vi "Main.vi"() -> ()   [LabVIEW 2018] (continued)
  # "(Shutter Off)"
  # "V_IF (0.5pi or -1.5pi)"
  # "V_IF (pi or -pi)"
  # "V_IF (1.5pi or -0.5pi)"
  # "Pixel width calibration:\n1. Move the cursor to a feature pixel that you can recognize\n2. Click \"Record X1\" to record the X coordinate\n\n \n3. Use \"X-\" or \"X+\" with \"XY Step\" of 30 um to move the image horizentally by 30 um\n4. Move the cursor to the same feature pixel\n5. Click \"Record X2\" to record the X coordinate again\n\n\n6. Click \"Pixel Width\" to calculate the pixel width (um/px)\n7. Input your desired pixel width (um/px) and the cooresponding \"XY Factor (1/V)\" will be calculated"
  # "Based on \"Desired Pixel Wdith (um)\""
  # "Going inside the sample (Z increase)"
  # "Z4\nAst45"
  # "Z5\nDef"
  # "Z6\nAst0"
  # "Z7\nTreY"
  # "Z8\nComX"
  # "Z9\nComY"
  # "Z10\nTreX"
  # "Z11\nTetY"
  # "Z12\nSAstY"
  # "Z13\nSAb3"
  # "Z14\nSAstX"
  # "Z15\nTetX"
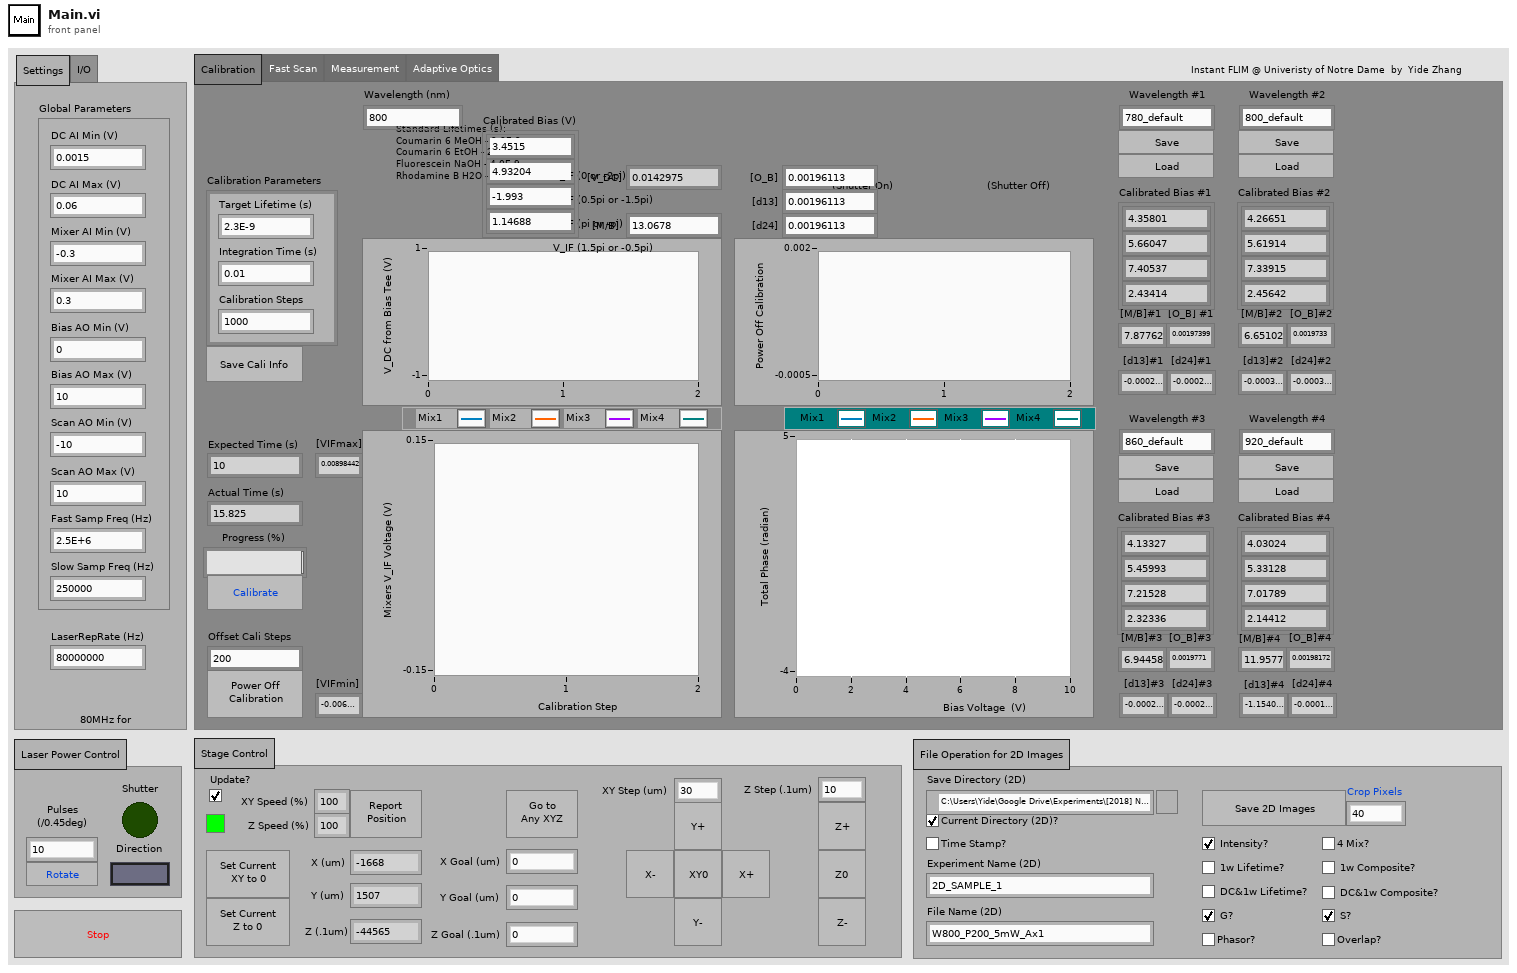
[diagram p1: front panel]
types:
  T1 = cluster{"DC AI Min (V)":dbl, "DC AI Max (V)":dbl, "Mixer AI Min (V)":dbl, "Mixer AI Max (V)":dbl, "Bias AO Min (V)":dbl, "Bias AO Max (V)":dbl, "Scan AO Min (V)":dbl, "Scan AO Max (V)":dbl, "Fast Samp Freq (Hz)":dbl, "Slow Samp Freq (Hz)":dbl}
  T2 = enum32{"Calibration", "Fast Scan", "Measurement", "Adaptive Optics"}
  T3 = cluster{"Target Lifetime (s)":dbl, "Integration Time (s)":dbl, "Calibration Steps":dbl}
  T4 = cluster{"Pixel Dwell Time (s)":dbl, "Pixel Size":dbl, "X Min (V)":dbl, "X Max (V)":dbl, "Y Min (V)":dbl, "Y Max (V)":dbl, "XY Factor (1/V)":dbl}
  T5 = enum16{"Nikon 40X NA 0.8 WD=3.5mm", "Olympus 25X NA 1.05 WD=2mm"}
  T6 = enum32{"Process", "Results", "Phasors", "Z-Stack", "Time-Lapse", "GSOS Process", "GSOS Results"}
  T7 = cluster{"X Values":dbl[], "Histogram: h(x)":i32[]}
  T8 = enum16{"fire", "rainbow", "gray", "inverse gray", "ice", "original"}
  T9 = cluster{bool[], dbl[], cluster{dbl, dbl}[], u32[]}
  T10 = enum16{"Intensity 3D", "1w Lifetime 3D", "DC&1w Lifetime 3D", "1w Composite 3D", "DC&1w Composite 3D", "Phasor 3D", "Overlap 3D"}
  T11 = enum16{"Mean Pixel Value", "Normalized Variance", "Mean Squared Pixel Value"}
  T12 = cluster{"Mixer AI Channel(s)":tag, "DC AI Channel(s)":tag, "Bias AO Channel(s) ":tag, "Scan AO Channel(s)":tag}
  T13 = enum32{"Calibration", "Fast Scan", "Measurement"}
  T14 = cluster{"DC AI task out":refnum<k21>, "Mixer AI task out":refnum<k21>, "Bias AO task out":refnum<k21>, "Scan AO task out":refnum<k21>}
  T15 = typedef "NI_LVConfig.lvlib/Config Data RefNum.ctl" = refnum<k1>
  T16 = typedef "LVBoundsTypeDef.ctl" = cluster{"Width":u32, "Height":u32}
  T17 = typedef "lveventtype.ctl" = enum32{"Null", "Timeout", "Annotation Menu Selection", "Annotation Menu Selection?", "App Instance Close", "App Instance Close?", "Autoscale Range Change", "Bookmark Info Change", "Cell Edit", "Cell Edit?", "Cursor Grab", "Cursor Grab?", "Cursor Menu Selection", "Cursor Menu Selection?", "Cursor Move", "Cursor Release", "Data Change", "Direction Change", "Display State Change", "Drag Ended", "Drag Enter", "Drag Leave", "Drag Over", "Drag Source Update", "Drag Starting", "Drag Starting?", "Drop", "Exec State Change", "Key Down", "Key Down?", "Key Repeat", "Key Repeat?", "Key Up", "Listbox Double Click", "Menu Activation?", "Menu Selection (App)", "Menu Selection? (App)", "Menu Selection (User)", "Mouse Down", "Mouse Down?", "Mouse Enter", "Mouse Leave", "Mouse Move", "Mouse Up", "Mouse Wheel", "NI Security User Change (App)", "Pane Size", "Panel Close", "Panel Close?", "Panel Resize", "Plot Attribute Change", "Scale Range Change", "Shortcut Menu Activation?", "Shortcut Menu Selection (App)", "Shortcut Menu Selection? (App)", "Shortcut Menu Selection (User)", "Tree Double Click", "Tree Drag", "Tree Drag?", "Tree Drop", "Tree Drop?", "Tree Item Close", "Tree Item Close?", "Tree Item Open", "Tree Item Open?", "User Event", "Value Change"}
  T18 = typedef "LVRectTypeDef.ctl" = cluster{"Left":i16, "Top":i16, "Right":i16, "Bottom":i16}
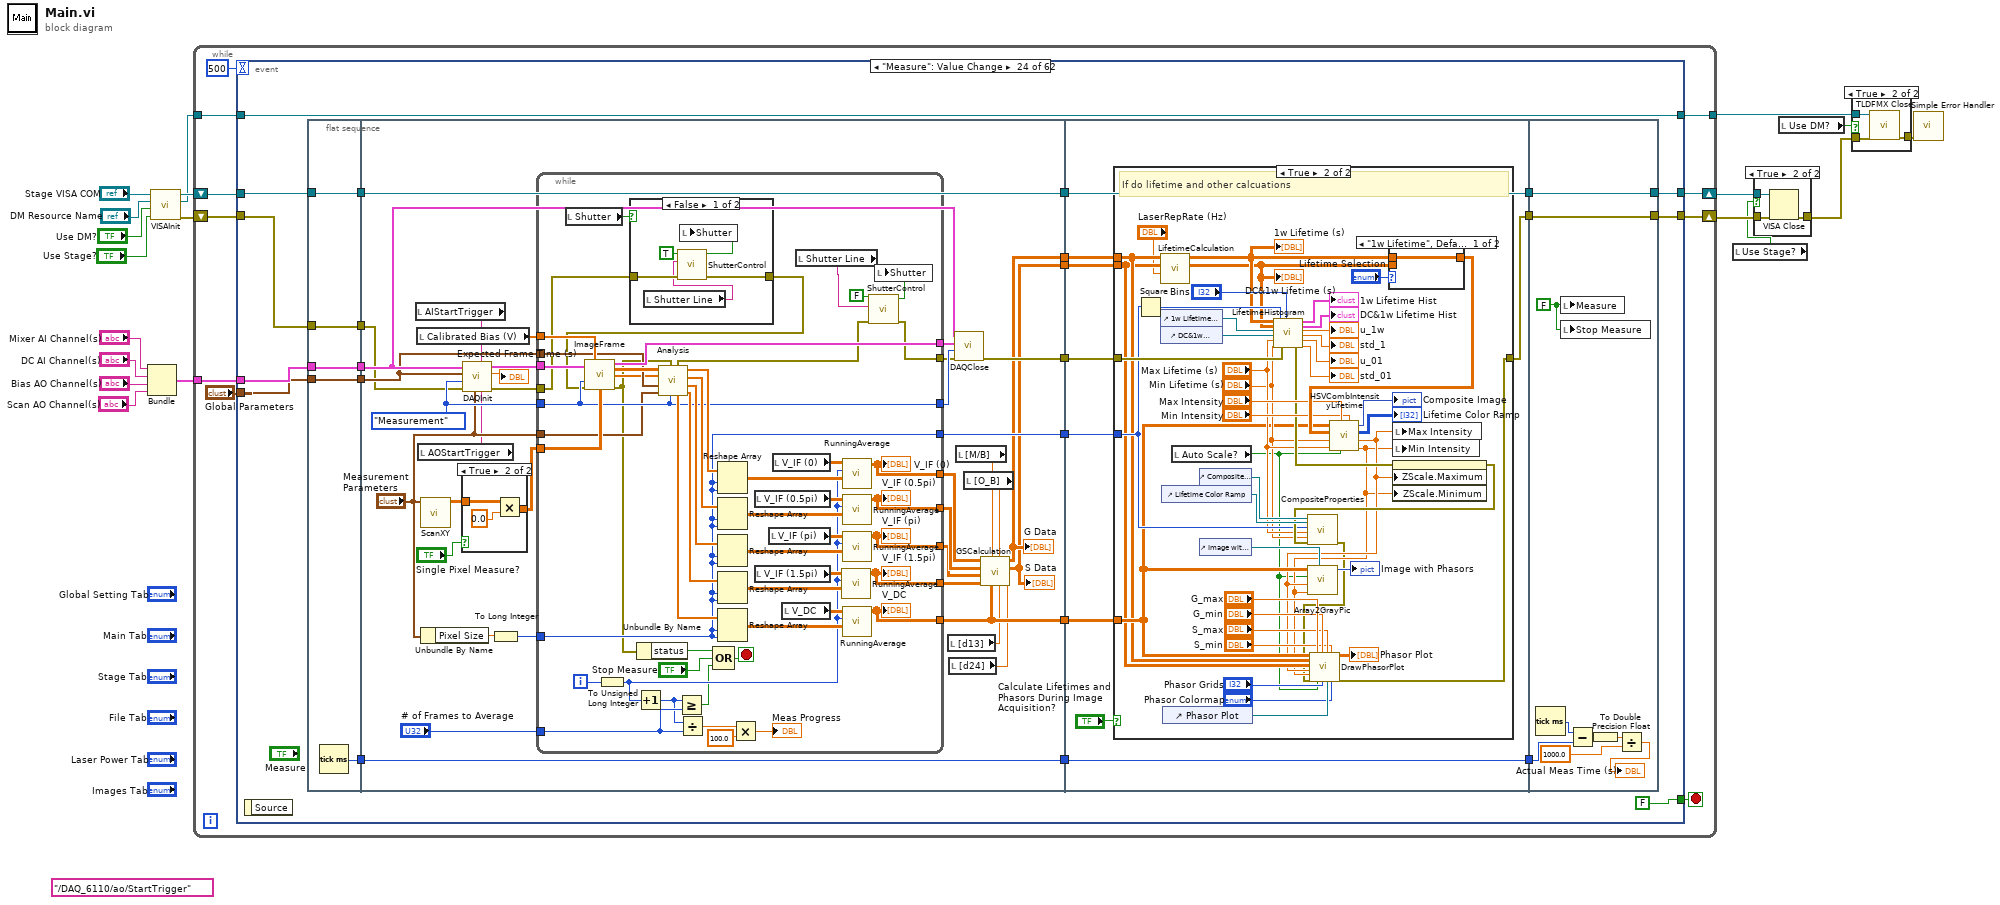
[diagram p0: block diagram]
diagram:
  (unwired) tag "/DAQ_6110/ao/StartTrigger" ("source")
  n1 = Bundle("Mixer AI Channel(s)"="Mixer AI Channel(s)", "DC AI Channel(s)"="DC AI Channel(s)", "Bias AO Channel(s)"="Bias AO Channel(s)", "Scan AO Channel(s)"="Scan AO Channel(s)") -> (w15:T12)  [unwired: 1 in]
  n2 = call "VISAInit.vi"("Use Stage?"="Use Stage?", "Use DM?"="Use DM?", "DM Resource Name"="DM Resource Name", "Stage Resource Name"="Stage VISA COM") -> ("error out"=w14:errorcluster, "DM Handle"=w10:refnum<visa-resource-name>, "Stage Resource"=w13:refnum<visa-resource-name>)  [unwired: 5 in]
  n3 = while {
    shift-right: [w24] -> w19
    shift-left: w13 -> [w29]
    shift-right: [w23] -> w18
    shift-left: w14 -> [w28]
    tunnel: w15 -> [w27]
    tunnel: w10 -> [w22]
    tunnel: [w21] -> w7
    stop <- w26 stop-if-true
    n4 = event shown="[23] \"Measure\": Value Change" {
      selector: _ -> [_ _ _ _ _ _ _ _ _ _ _ _ _ _ _ _ _ _ _ _ _ _ _ _ _ _ _ _ _ _ _ _ _ _ _ _ _ _ _ _ _ _ _ _ _ _ _ _ _ _ _ _ _ _ _ _ _ _ _ _ _ _]
      dyn-events: _ -> [_ _ _ _ _ _ _ _ _ _ _ _ _ _ _ _ _ _ _ _ _ _ _ _ _ _ _ _ _ _ _ _ _ _ _ _ _ _ _ _ _ _ _ _ _ _ _ _ _ _ _ _ _ _ _ _ _ _ _ _ _ _]
      timeout: 500 -> [_ _ _ _ _ _ _ _ _ _ _ _ _ _ _ _ _ _ _ _ _ _ _ _ _ _ _ _ _ _ _ _ _ _ _ _ _ _ _ _ _ _ _ _ _ _ _ _ _ _ _ _ _ _ _ _ _ _ _ _ _ _]
      tunnel: [FALSE ("Shutter") FALSE ("Shutter") FALSE ("Shutter") FALSE ("Shutter") FALSE ("Shutter") FALSE ("Shutter") FALSE ("Shutter") FALSE ("Shutter") FALSE ("Shutter") FALSE ("Shutter") FALSE ("Shutter") FALSE ("Shutter") FALSE ("Shutter") FALSE ("Shutter") FALSE ("Shutter") _ FALSE ("Shutter") _ _ _ _ FALSE ("Shutter") _ FALSE ("Shutter") FALSE ("Shutter") FALSE ("Shutter") FALSE ("Shutter") FALSE ("Shutter") FALSE ("Shutter") FALSE ("Shutter") FALSE ("Shutter") FALSE ("Shutter") FALSE ("Shutter") FALSE ("Shutter") FALSE ("Shutter") FALSE ("Shutter") FALSE ("Shutter") FALSE ("Shutter") FALSE ("Shutter") FALSE ("Shutter") FALSE ("Shutter") FALSE ("Shutter") FALSE ("Shutter") FALSE ("Shutter") "Stop" FALSE ("Shutter") FALSE ("Shutter") FALSE ("Shutter") FALSE ("Shutter") FALSE ("Shutter") FALSE ("Shutter") FALSE ("Shutter") FALSE ("Shutter") FALSE ("Shutter") FALSE ("Shutter") FALSE ("Shutter") FALSE ("Shutter") FALSE ("Shutter") FALSE ("Shutter") FALSE ("Shutter") FALSE ("Shutter") FALSE ("Shutter")] -> w26
      tunnel: w29 -> [w37 w94 w123 w284 w373 w395 w405 w415 w423 w435 w445 w455 w465 w482 w577 w610 w620 w668 w682 w719 w837 w924 w997 w1132 w1305 w1381 w1530 w1688 w1712 w1751 w1818 w1859 w1889 w2052 w2117 w2160 w2208 w2263 w2350 w2404 w2513 w2528 w2537 w2546 w2557 w2565 w2590 w2615 w2640 w2663 w2688 w2715 w2734 w2753 w2780 w2799 w2817 w2866 w2870 w2882 w2888 w2907]
      tunnel: w28 -> [w38 w92 w122 w281 w374 w394 w404 w414 w422 w434 w444 w454 w464 w474 w572 w607 w623 w664 w676 w715 w836 w919 w993 w1121 w1302 w1380 w1506 w1682 w1703 w1742 w1782 w1826 w1918 w2043 w2114 w2135 w2185 w2239 w2351 w2417 w2466 w2527 w2536 w2545 w2556 w2564 w2589 w2614 w2639 w2662 w2687 w2714 w2733 w2752 w2779 w2798 w2818 w2864 w2872 w2881 w2887 w2906]
      tunnel: [w34 w94 w121 w283 w373 w395 w405 w415 w423 w435 w445 w455 w465 w481 w577 w610 w620 w668 w682 w719 w837 w924 w997 w1117 w1304 w1367 w1530 w1688 w1712 w1751 w1818 w1859 w1889 w2052 w2117 w2160 w2208 w2263 w2350 w2404 w2513 w2528 w2537 w2546 w2557 w2560 w2585 w2610 w2635 w2660 w2685 w2710 w2729 w2748 w2777 w2796 w2816 w2866 w2870 w2882 w2888 w2907] -> w24
      tunnel: [w33 w91 w115 w280 w351 w394 w404 w414 w422 w434 w444 w454 w464 w472 w575 w605 w621 w662 w678 w721 w833 w914 w996 w1123 w1301 w1365 w1520 w1660 w1702 w1741 w1784 w1825 w1897 w2020 w2113 w2124 w2173 w2228 w2319 w2405 w2484 w2527 w2535 w2544 w2555 w2559 w2584 w2609 w2634 w2659 w2684 w2709 w2728 w2747 w2778 w2797 w2815 w2863 w2871 w2881 w2887 w2906] -> w23
      tunnel: w27 -> [_ _ w119 w279 _ _ _ _ _ _ _ _ _ w480 _ _ _ _ _ _ _ _ _ w1126 _ _ _ _ _ _ _ _ _ _ _ _ _ _ _ _ _ _ _ _ _ _ _ _ _ _ _ _ _ _ _ _ _ _ _ _ _ _]
      tunnel: "Global Parameters" -> [_ _ w117 w278 _ _ _ _ _ _ _ _ _ w479 _ _ _ _ _ _ _ _ _ w1124 _ _ _ _ _ _ _ _ _ _ _ _ _ _ _ _ _ _ _ _ _ _ _ _ _ _ _ _ _ _ _ _ _ _ _ _ _ _]
      tunnel: [w36 w85 w101 w276 w340 w392 w399 w409 w419 w429 w439 w449 w459 w471 w576 w606 w619 w667 w683 w717 w834 w917 w995 w1111 w1300 w1364 w1495 w1659 w1701 w1740 w1777 w1822 w1864 w2007 w2098 w2120 w2168 w2216 w2270 w2383 w2435 w2525 w2533 w2541 w2548 w2563 w2588 w2613 w2638 w2665 w2690 w2713 w2732 w2751 w2776 w2795 w2814 w2862 w2868 w2874 w2884 w2894] -> w21
      tunnel: w22 -> [w36 w85 w101 w276 w340 w392 w399 w409 w419 w429 w439 w449 w459 w471 w573 w608 w622 w667 w683 w718 w835 w918 w994 w1111 w1300 w1364 w1495 w1659 w1701 w1740 w1777 w1822 w1864 w2007 w2098 w2120 w2168 w2216 w2270 w2383 w2435 w2525 w2533 w2541 w2548 w2563 w2588 w2613 w2638 w2665 w2690 w2713 w2732 w2751 w2776 w2795 w2814 w2862 w2868 w2874 w2884 w2894]
      event Timeout {
        n5 = event-data() -> ()  [unwired: 1 in, 1 out]
        n6 = local read "Use Stage?"() -> (w30:bool)
        n7 = And(x="Update?", y=w30) -> (x .and. y?=w31:bool)
        n8 = case shown="True" w31 {
          tunnel: w38 -> [w39 w66]
          tunnel: w37 -> [w40 w65]
          tunnel: [w40 w41] -> w34
          tunnel: [w39 w42] -> w33
          frame False {
          }
          frame True {
            n9 = local read "Timeout Indicator"() -> (w46:bool)
            n10 = VISA Write(VISA resource name=w65, write buffer="P" ("string"), error in (no error)=w66) -> (VISA resource name out=w74:refnum<visa-resource-name>, error out=w73:errorcluster)  [unwired: 1 out]
            n11 = Not(x=w46) -> (.not. x?=→"Timeout Indicator":bool)
            n12 = VISA Read(VISA resource name=w74, byte count=u32 256, error in (no error)=w73) -> (VISA resource name out=w52:refnum<visa-resource-name>, read buffer=w79:string, error out=w54:errorcluster)  [unwired: 1 out]
            n13 = Search/Split String(string=w79, search string/char (-)=",") -> (substring before match=→"X (um)":string, match + rest of string=w71:string)  [unwired: 1 in, 1 out]
            n14 = Search/Split String(string=w71, search string/char (-)=",", offset (0)=1) -> (substring before match=w68:string, match + rest of string=w81:string)  [unwired: 1 out]
            n15 = VISA Clear(VISA resource name=w52, error in (no error)=w54) -> (VISA resource name out=w51:refnum<visa-resource-name>, error out=w53:errorcluster)
            n16 = String Subset(string=w68, offset (0)=1) -> (substring=→"Y (um)":string)  [unwired: 1 in]
            n17 = String Subset(string=w81, offset (0)=1) -> (substring=→"Z (.1um)":string)  [unwired: 1 in]
            n18 = VISA Write(VISA resource name=w51, write buffer="O" ("string"), error in (no error)=w53) -> (VISA resource name out=w62:refnum<visa-resource-name>, error out=w63:errorcluster)  [unwired: 1 out]
            n19 = VISA Read(VISA resource name=w62, byte count=u32 256, error in (no error)=w63) -> (VISA resource name out=w50:refnum<visa-resource-name>, read buffer=→"XY Speed (%)":string, error out=w49:errorcluster)  [unwired: 1 out]
            n20 = VISA Clear(VISA resource name=w50, error in (no error)=w49) -> (VISA resource name out=w48:refnum<visa-resource-name>, error out=w47:errorcluster)
            n21 = VISA Write(VISA resource name=w48, write buffer="OF" ("string"), error in (no error)=w47) -> (VISA resource name out=w57:refnum<visa-resource-name>, error out=w58:errorcluster)  [unwired: 1 out]
            n22 = VISA Read(VISA resource name=w57, byte count=u32 256, error in (no error)=w58) -> (VISA resource name out=w44:refnum<visa-resource-name>, read buffer=→"Z Speed (%)":string, error out=w43:errorcluster)  [unwired: 1 out]
            n23 = VISA Clear(VISA resource name=w44, error in (no error)=w43) -> (VISA resource name out=w41:refnum<visa-resource-name>, error out=w42:errorcluster)
          }
        }
      }
      event Panel Close? {
        n24 = event-data() -> ()  [unwired: 1 in, 1 out]
        n25 = call "ShutterControl.vi"("error in"=w92, "Shutter Line"="Shutter Line", "Shutter"=FALSE) -> ("error out"=w91:errorcluster, "Status Indicator"=w90:bool)  [unwired: 7 in]
        n26 = local write "Shutter"(w90) -> ()
        n27 = Two Button Dialog(message="Do you really want to exit?") -> (T button?=w96:bool)  [unwired: 2 in]
        n28 = local write "Meas Progress"(0.0 ("Fast Scan Progress")) -> ()
        n29 = local write "Fast Scan Progress"(0.0 ("Fast Scan Progress")) -> ()
        n30 = local write "Measure"(FALSE ("Fast Scan")) -> ()
        n31 = local write "Fast Scan"(FALSE ("Fast Scan")) -> ()
        n32 = Not(x=w96) -> (.not. x?=w95:bool)
        n33 = event-data("Discard?"=w95) -> ()  [unwired: 1 in, 1 out]
      }
      event "Calibrate": Value Change {
        n34 = event-data() -> ()  [unwired: 1 in, 1 out]
        n35 = flat-sequence {
          tunnel: w123 -> [w132]
          tunnel: [w132] -> w127
          tunnel: [w131] -> w126
          tunnel: w122 -> [w131]
          tunnel: [w130] -> w125
          tunnel: [w129] -> w120
          tunnel: w119 -> [w129]
          tunnel: w117 -> [w128]
          tunnel: [w128] -> w118
          tunnel: w127 -> [w192]
          tunnel: [w192] -> w124
          tunnel: w126 -> [w191]
          tunnel: w125 -> [w154]
          tunnel: w120 -> [w163]
          tunnel: w118 -> [w183]
          tunnel: [w164] -> w116
          tunnel: [w183] -> w114
          tunnel: ["Calibration Parameters"] -> w113
          tunnel: [w181] -> w112
          tunnel: [w180] -> w111
          tunnel: [w177] -> w110
          tunnel: [w176] -> w109
          tunnel: [w175] -> w108
          tunnel: [w171] -> w107
          tunnel: [w155] -> w106
          tunnel: [w154] -> w103
          tunnel: [w142] -> w99
          tunnel: [w141] -> w98
          tunnel: w124 -> [w261]
          tunnel: w116 -> [w260]
          tunnel: w114 -> [w259]
          tunnel: w113 -> [w258]
          tunnel: w112 -> [w254]
          tunnel: w111 -> [w253]
          tunnel: w110 -> [w252]
          tunnel: w109 -> [w251]
          tunnel: w108 -> [w250]
          tunnel: w107 -> [w248]
          tunnel: w106 -> [w243]
          tunnel: [w261] -> w105
          tunnel: [w260] -> w104
          tunnel: w103 -> [w244]
          tunnel: [w244] -> w102
          tunnel: w99 -> [w241]
          tunnel: w98 -> [w240]
          tunnel: [w271] -> w115
          tunnel: [w272] -> w121
          tunnel: w105 -> [w272]
          tunnel: w104 -> [w271]
          tunnel: w102 -> [w265]
          frame #0 {
            n36 = Tick Count (ms)() -> (millisecond timer value=w130:u32)
          }
          frame #1 {
            w145 = 0.0
            w189 = T13."Calibration" ("Main Tab")
            n37 = flat-sequence {
              tunnel: [w201] -> w152
              tunnel: w156 -> [w201]
              frame #0 {
                n38 = Wait (ms)(milliseconds to wait=u32 100) -> ()  [unwired: 1 out]
              }
            }
            n39 = call "DAQInit.vi"("AOStartTrigger"="AOStartTrigger", "AIStartTrigger"="AIStartTrigger", "Calibration Parameters"="Calibration Parameters", "error in"=w191, "Functions"=w189, "Global Parameters"=w183, "DAQ Channels"=w163) -> ("error out"=w185:errorcluster, "Expected Time (s)"=→"Expected Time (s)":dbl, "Tasks Out"=w162:T14)  [unwired: 2 in]
            n40 = Unbundle By Name("Calibration Parameters") -> ("Calibration Steps"=w188:dbl)
            n41 = local read "Shutter Line"() -> (w135:tag)
            n42 = call "ShutterControl.vi"("error in"=w185, "Shutter Line"=w135, "Shutter"=TRUE) -> ("error out"=w167:errorcluster, "Status Indicator"=w179:bool)  [unwired: 7 in]
            n43 = local write "Shutter"(w179) -> ()
            n44 = flat-sequence {
              tunnel: [w207] -> w166
              tunnel: w167 -> [w207]
              frame #0 {
                n45 = Wait (ms)(milliseconds to wait=u32 100) -> ()  [unwired: 1 out]
              }
            }
            n46 = while {
              tunnel: w162 -> [w234]
              tunnel: w166 -> [w233]
              tunnel: w189 -> [w217]
              tunnel: "Calibration Parameters" -> [w231]
              tunnel: w183 -> [w229]
              tunnel: w188 -> [w230]
              tunnel: [w223] -> w180 mode=concatenating
              tunnel: [w226] -> w165
              tunnel: [w228] -> w153
              tunnel: [w217] -> w187
              tunnel: [w218] -> w181 mode=indexing
              tunnel: [w221] -> w177 mode=concatenating
              tunnel: [w220] -> w176 mode=concatenating
              tunnel: [w219] -> w175 mode=concatenating
              tunnel: [w216] -> w168 mode=concatenating
              i -> [w238]
              stop <- w224 stop-if-true
              n47 = To Double Precision Float(number=w238) -> (double precision float=w212:dbl)
              n48 = call "ImageFrame.vi"("Tasks In"=w234, "Global Parameters"=w229, "Calibration Parameters"=w231, "Functions"=w217, "error in"=w233, "index"=w212) -> ("Tasks Out"=w228:T14, "Mixer AI Channels Data"=w215:dbl[][], "DC AI Channel Date"=w214:dbl[], "Bias Voltage"=w218:dbl, "error out"=w226:errorcluster)  [unwired: 5 in]
              n49 = Increment(x=w212) -> (x+1=w213:dbl)
              n50 = call "Analysis.vi"("Functions"=w217, "DC AI Channel Data"=w214, "Mixer AI Channels Data"=w215) -> ("AI Mix4 Data"=w219:dbl[], "AI Mix3 Data"=w220:dbl[], "AI Mix2 Data"=w221:dbl[], "AI Mix1 Data"=w223:dbl[], "AI DC Data"=w216:dbl[])  [unwired: 3 in, 1 out]
              "Calibration AI  Signals (Integrated) 2" <- w216
              n51 = Unbundle By Name(w226) -> ("status"=w227:bool)
              n52 = Greater Or Equal?(x=w213, y=w230) -> (x >= y?=w225:bool)
              n53 = Divide(x=w213, y=w230) -> (x/y=w237:dbl)
              n54 = Build Array(w223, w221, w220, w219) -> (→"Calibration AI  Signals (Integrated)":dbl[][])
              n55 = Multiply(x=w237, y=100.0) -> (x*y=w235:dbl)
              n56 = Compound Arithmetic op=OR(w227, w225) -> (w224:bool)
              n57 = To Unsigned Byte Integer(number=w235) -> (unsigned 8bit integer=→"Calibrate Progress":u8)
            }
            n58 = call "PowerOffCalibration.vi"("Tasks In"=w153, "Offset Cali Steps"="Offset Cali Steps", "error in"=w152) -> ("Tasks Out"=w150:T14, "V_DC Array"=w140:dbl[], "d13 Array"=w139:dbl[], "d24 Array"=w138:dbl[], "error out"=w149:errorcluster)  [unwired: 8 in]
            n59 = Build Array(w140, w139, w138) -> (→"Power Off Voltages":dbl[][])
            n60 = local read "Shutter Line"() -> (w136:tag)
            n61 = call "ShutterControl.vi"("error in"=w165, "Shutter Line"=w136, "Shutter"=FALSE) -> ("error out"=w156:errorcluster, "Status Indicator"=w178:bool)  [unwired: 7 in]
            n62 = local write "Shutter"(w178) -> ()
            n63 = for {
              tunnel: w140 -> [w205] mode=indexing
              shift-right: [w203] -> w157
              shift-left: 0.0 -> [w204]
              tunnel: [w202] -> w160
              i -> [w202]
              n64 = Add(x=w205, y=w204) -> (x+y=w203:dbl)
            }
            n65 = for {
              tunnel: w168 -> [w211] mode=indexing
              shift-right: [w209] -> w174
              shift-left: 0.0 -> [w210]
              tunnel: [w208] -> w170
              i -> [w208]
              n66 = Add(x=w211, y=w210) -> (x+y=w209:dbl)
            }
            n67 = for {
              tunnel: w139 -> [w199] mode=indexing
              shift-right: [w197] -> w148
              shift-left: w145 -> [w198]
              tunnel: [w196] -> w146
              tunnel: w138 -> [w195] mode=indexing
              shift-right: [w193] -> w144
              shift-left: w145 -> [w194]
              i -> [w196]
              n68 = Add(x=w199, y=w198) -> (x+y=w197:dbl)
              n69 = Add(x=w195, y=w194) -> (x+y=w193:dbl)
            }
            n70 = Increment(x=w146) -> (x+1=w147:i32)
            n71 = Increment(x=w160) -> (x+1=w161:i32)
            n72 = Increment(x=w170) -> (x+1=w169:i32)
            n73 = To Double Precision Float(number=w147) -> (double precision float=w143:dbl)
            n74 = To Double Precision Float(number=w161) -> (double precision float=w158:dbl)
            n75 = To Double Precision Float(number=w169) -> (double precision float=w173:dbl)
            n76 = Divide(x=w148, y=w143) -> (x/y=w142:dbl)
            n77 = Divide(x=w157, y=w158) -> (x/y=w155:dbl)
            n78 = Divide(x=w144, y=w143) -> (x/y=w141:dbl)
            n79 = Divide(x=w174, y=w173) -> (x/y=w171:dbl)
            n80 = call "DAQClose.vi"("error in"=w149, "Functions"=w187, "Tasks In"=w150, "DAQ Channels"=w163) -> ("error out"=w164:errorcluster)  [unwired: 7 in]
          }
          frame #2 {
            n81 = local read "LaserRepRate (Hz)"() -> (w239:dbl)
            n82 = local write "[d13]"(w241) -> ()
            n83 = local write "[d24]"(w240) -> ()
            n84 = call "PhaseCalibration.vi"("Global Parameters"=w259, "Bias Voltages"=w254, "LaserRepRate"=w239, "Calibration Parameters"=w258, "Mixer1 Values"=w253, "Mixer2 Values"=w252, "Mixer3 Values"=w251, "Mixer4 Values"=w250, "[V_DC]"=w248, "[O_B]"=w243) -> ("Mixer Phases"=→"Mixer Phases":cluster{"Bias voltage":dbl[], dbl[]}[], "Calibrated Bias Voltages"=w247:dbl[], "[M/B]"=w242:dbl, "[V_IF_max]"=→"[VIFmax]":dbl, "[V_IF_min]"=→"[VIFmin]":dbl)  [unwired: 1 in]
            n85 = local write "[O_B]"(w243) -> ()
            n86 = Greater?(x=w247, y=10.0) -> (0:w256:bool[])
            n87 = local write "[M/B]"(w242) -> ()
            n88 = Or Array Elements(Boolean array=w256) -> (logical OR=w255:bool)
            n89 = case shown="False" w255 {
              tunnel: w247 -> [w262 _]
              frame False {
                n90 = local write "Calibrated Bias (V)"(w262) -> ()
              }
              frame True {
                n91 = One Button Dialog(message="Calibration failed.\nVoltage out of bound.\nPlease re-calibrate.") -> ()  [unwired: 1 in, 1 out]
              }
            }
            "[V_DC]" <- w248
          }
          frame #3 {
            n92 = Tick Count (ms)() -> (millisecond timer value=w267:u32)
            n93 = Subtract(x=w267, y=w265) -> (x-y=w268:u32)
            n94 = local write "Calibrate"(FALSE ("Fast Scan")) -> ()
            n95 = To Double Precision Float(number=w268) -> (double precision float=w269:dbl)
            n96 = Divide(x=w269, y=1000.0) -> (x/y=→"Actual Time (s)":dbl)
          }
        }
      }
      event "PowerOffCalibration": Value Change {
        n97 = event-data() -> ()  [unwired: 1 in, 1 out]
        n98 = flat-sequence {
          tunnel: [w321] -> w285
          tunnel: w284 -> [w321]
          tunnel: [w306] -> w282
          tunnel: w281 -> [w318]
          tunnel: w279 -> [w308]
          tunnel: w278 -> [w316]
          tunnel: [w309] -> w277
          tunnel: [w294] -> w274
          tunnel: [w293] -> w273
          tunnel: w285 -> [w338]
          tunnel: [w338] -> w283
          tunnel: w282 -> [w337]
          tunnel: [w337] -> w280
          tunnel: w277 -> [w336]
          tunnel: w274 -> [w334]
          tunnel: w273 -> [w333]
          frame #0 {
            w297 = 0.0
            w307 = T13."Calibration" ("Main Tab")
            n99 = local read "Calibration Parameters"() -> (w315:T3)
            n100 = local read "AIStartTrigger"() -> (w287:tag)
            n101 = local read "AOStartTrigger"() -> (w286:tag)
            n102 = call "DAQInit.vi"("AOStartTrigger"=w286, "AIStartTrigger"=w287, "Calibration Parameters"=w315, "error in"=w318, "Functions"=w307, "Global Parameters"=w316, "DAQ Channels"=w308) -> ("error out"=w317:errorcluster, "Tasks Out"=w304:T14)  [unwired: 2 in, 1 out]
            n103 = local read "Shutter Line"() -> (w288:tag)
            n104 = call "ShutterControl.vi"("error in"=w317, "Shutter Line"=w288, "Shutter"=FALSE) -> ("error out"=w305:errorcluster, "Status Indicator"=w319:bool)  [unwired: 7 in]
            n105 = local write "Shutter"(w319) -> ()
            n106 = local read "Offset Cali Steps"() -> (w303:dbl)
            n107 = call "PowerOffCalibration.vi"("Tasks In"=w304, "Offset Cali Steps"=w303, "error in"=w305) -> ("Tasks Out"=w302:T14, "V_DC Array"=w291:dbl[], "d13 Array"=w290:dbl[], "d24 Array"=w289:dbl[], "error out"=w301:errorcluster)  [unwired: 8 in]
            n108 = Build Array(w291, w290, w289) -> (w292:dbl[][])
            n109 = local write "Power Off Voltages"(w292) -> ()
            n110 = for {
              tunnel: w291 -> [w332] mode=indexing
              shift-right: [w330] -> w310
              shift-left: 0.0 -> [w331]
              tunnel: [w329] -> w313
              i -> [w329]
              n111 = Add(x=w332, y=w331) -> (x+y=w330:dbl)
            }
            n112 = for {
              tunnel: w290 -> [w328] mode=indexing
              shift-right: [w326] -> w300
              shift-left: w297 -> [w327]
              tunnel: [w325] -> w298
              tunnel: w289 -> [w324] mode=indexing
              shift-right: [w322] -> w296
              shift-left: w297 -> [w323]
              i -> [w325]
              n113 = Add(x=w328, y=w327) -> (x+y=w326:dbl)
              n114 = Add(x=w324, y=w323) -> (x+y=w322:dbl)
            }
            n115 = Increment(x=w298) -> (x+1=w299:i32)
            n116 = Increment(x=w313) -> (x+1=w314:i32)
            n117 = call "DAQClose.vi"("error in"=w301, "Functions"=w307, "Tasks In"=w302, "DAQ Channels"=w308) -> ("error out"=w306:errorcluster)  [unwired: 7 in]
            n118 = To Double Precision Float(number=w299) -> (double precision float=w295:dbl)
            n119 = To Double Precision Float(number=w314) -> (double precision float=w311:dbl)
            n120 = Divide(x=w300, y=w295) -> (x/y=w294:dbl)
            n121 = Divide(x=w296, y=w295) -> (x/y=w293:dbl)
            n122 = Divide(x=w310, y=w311) -> (x/y=w309:dbl)
          }
          frame #1 {
            n123 = local write "[O_B]"(w336) -> ()
            n124 = local write "[d13]"(w334) -> ()
            n125 = local write "[d24]"(w333) -> ()
            n126 = local write "PowerOffCalibration"(FALSE ("Re-Calibrate O")) -> ()
          }
        }
      }
      event "Save Calibration Info": Value Change {
        w345 = "Calibration" ("string")
        n127 = event-data() -> ()  [unwired: 1 in, 1 out]
        n128 = Current VI's Path() -> (path=w372:path)
        n129 = Strip Path(path=w372) -> (stripped path=w375:path)  [unwired: 1 out]
        n130 = local read "Mixer Phases"() -> (w350:cluster{"X":dbl[], "Y":dbl[]}[])
        n131 = Concatenate Strings(w345, "_" ("string"), "Wavelength (nm)", "nm" ("string")) -> (w342:string)
        n132 = Build Path(base path=w375, name or relative path=w345) -> (appended path=w376:path)
        n133 = call <vilib>:"Check if File or Folder Exists.vi"("error in (no error)"=w374, "path"=w376) -> ("error out"=w378:errorcluster, "file or folder exists?"=w377:bool, "dup path"=w379:path)  [unwired: 7 in]
        n134 = case shown="False" w377 {
          tunnel: w378 -> [w383 w384]
          tunnel: [w382 w384] -> w369
          tunnel: [w381 w385] -> w364
          tunnel: w379 -> [w380 w385]
          frame False {
            n135 = Create Folder(path (use dialog)=w380, error in=w383) -> (created path=w381:path, error out=w382:errorcluster)  [unwired: 1 in, 1 out]
          }
          frame True {
          }
        }
        n136 = property on="Calibration AI  Signals (Integrated)" class="WFChart (strict)"() -> ("History Data"=w371:dbl[][])  [unwired: 2 in, 2 out]